vi "pharmaBot_v0.019.vi"() -> ()   [LabVIEW 2015] (continued)
            n1468 = call "get_XYZ.vi"("Actuator cluster in"=w1988) -> ("X pos (steps)"=w1996:i32, "Y pos (steps)"=w1995:i32, "Z pos (steps)"=w1994:i32)  [unwired: 10 in, 2 out]
            n1469 = Build Array(w1996, w1995, w1994) -> (w1993:i32[])
            n1470 = flat-sequence {
              tunnel: w1993 -> [w2006]
              tunnel: w1989 -> [w2005]
              frame #0 {
                n1471 = local read "location above baths"() -> (w2004:bool)
                n1472 = local read "wash bath location"() -> (w2002:bool)
                n1473 = local read "cleaning bath location"() -> (w2003:bool)
                n1474 = case shown="True" w2004 {
                  tunnel: w2006 -> [_ w2015]
                  tunnel: w2005 -> [_ w2016]
                  frame False {
                  }
                  frame True {
                    n1475 = case shown="\"manipulator 1\", Default" w2016 {
                      tunnel: w2015 -> [w2017 w2018]
                      frame "manipulator 1", Default {
                        n1476 = local write "loc above baths 1"(w2017) -> ()
                      }
                      frame "manipulator 2" {
                        n1477 = local write "loc above baths 2"(w2018) -> ()
                      }
                    }
                  }
                }
                n1478 = case shown="True" w2003 {
                  tunnel: w2006 -> [_ w2011]
                  tunnel: w2005 -> [_ w2012]
                  frame False {
                  }
                  frame True {
                    n1479 = case shown="\"manipulator 2\"" w2012 {
                      tunnel: w2011 -> [w2013 w2014]
                      frame "manipulator 1", Default {
                        n1480 = local write "cleaning bath loc 1"(w2013) -> ()
                      }
                      frame "manipulator 2" {
                        n1481 = local write "cleaning bath loc 2"(w2014) -> ()
                      }
                    }
                  }
                }
                n1482 = case shown="True" w2002 {
                  tunnel: w2006 -> [_ w2007]
                  tunnel: w2005 -> [_ w2008]
                  frame False {
                  }
                  frame True {
                    n1483 = case shown="\"manipulator 2\"" w2008 {
                      tunnel: w2007 -> [w2009 w2010]
                      frame "manipulator 1", Default {
                        n1484 = local write "wash bath loc 1"(w2009) -> ()
                      }
                      frame "manipulator 2" {
                        n1485 = local write "wash bath loc 2"(w2010) -> ()
                      }
                    }
                  }
                }
              }
              frame #1 {
                # "calculate \"above wash bath\" and \"above clean bath\" here\nin the future"
              }
            }
          }
        }
      }
      event "pipette autofocus": Value Change {
        n1486 = event-data() -> ("OldVal"=w2020:bool)  [unwired: 1 in, 5 out]
        n1487 = case shown="True" w2020 {
          tunnel: w2022 -> [_ w2039]
          tunnel: w2021 -> [_ w2038]
          frame False {
          }
          frame True {
            n1488 = local read "which manipulator to autofocus"() -> (w2024:T8)
            n1489 = case shown="\"manipulator 1\", Default" w2024 {
              tunnel: w2039 -> [w2076 w2081 w2083 w2085]
              tunnel: [w2075 w2080 w2082 w2084] -> w2037
              tunnel: [w2074 w2079 _ _] -> w2032
              tunnel: [w2073 w2078 _ _] -> w2031
              tunnel: [w2072 w2077 _ _] -> w2030
              frame "manipulator 1", Default {
                n1490 = local read "pipette 1 template"() -> (w2072:T10)
                n1491 = local read "found pipette 1"() -> (w2074:T10)
                n1492 = Unbundle By Name(w2076) -> ("manip 1"=w2075:refnum<vi>)
                n1493 = local read "manip 1 position"() -> (w2073:T23)
              }
              frame "manipulator 2" {
                n1494 = local read "pipette 2 template"() -> (w2077:T10)
                n1495 = local read "manip 2 position"() -> (w2078:T23)
                n1496 = Unbundle By Name(w2081) -> ("manip 2"=w2080:refnum<vi>)
                n1497 = local read "found pipette 2"() -> (w2079:T10)
              }
              frame "manipulator 3" {
                n1498 = Unbundle By Name(w2083) -> ("manip 3"=w2082:refnum<vi>)
              }
              frame "manipulator 4" {
                n1499 = Unbundle By Name(w2085) -> ("manip 4"=w2084:refnum<vi>)
              }
            }
            n1500 = call "get_screenCenter.vi"("image"=w2038) -> ("screen center (px)"=w2033:i32[])  [unwired: 10 in]
            n1501 = property class="Clust (strict)"(reference=w2037) -> (error out=w2028:errorcluster, "Value"=w2036:T25)  [unwired: 1 in, 1 out]
            n1502 = Unbundle By Name(w2036) -> ("actuator"=w2035:T26)
            n1503 = local read "pipette match score"() -> (w2034:sgl)
            n1504 = property on="tip found?" class="Bool (strict)"(error in=w2028, "Value"=FALSE ("tip found?")) -> (error out=w2027:errorcluster)  [unwired: 1 in, 1 out]
            n1505 = for {
              N: 1 -> [_]
              tunnel: w2033 -> [w2070]
              tunnel: [w2065] -> _
              tunnel: [w2066] -> _
              tunnel: w2035 -> [w2061]
              tunnel: w2027 -> [w2060]
              tunnel: w2039 -> [w2059]
              tunnel: w2024 -> [w2058]
              tunnel: w2038 -> [w2057]
              tunnel: w2030 -> [w2056]
              tunnel: w2032 -> [w2054]
              tunnel: [w2051] -> w2023
              tunnel: w2034 -> [w2048]
              tunnel: w2031 -> [w2053]
              tunnel: [w2043] -> w2025
              i -> [w2046]
              n1506 = call "Time Delay"("error in (no error)"=w2060, "Delay Time (s)"=1.0) -> ("error out"=w2063:errorcluster)  [unwired: 9 in]
              n1507 = Multiply(x=w2046, y=100) -> (x*y=w2050:i32)
              n1508 = Add(x=w2050, y=w2048) -> (x+y=w2047:sgl)
              n1509 = call "find_pipetteTip_v5.vi"("manip position"=w2053, "slice view"=w2057, "error in"=w2063, "pipette match score"=w2047, "pipette template"=w2056, "pipette in"=w2061) -> ("error out"=w2067:errorcluster, "tip found?"=w2051:bool, "screen tip location (px)"=w2052:i32[], "pipette out"=w2062:T26, "Score"=w2042:sgl, "found"=w2055:T10)
              n1510 = Subtract(x=w2070, y=w2052) -> (x-y=w2071:i32[])
              n1511 = call <vilib>:"Clear Errors.vi"("error in (no error)"=w2067) -> ("error out"=w2044:errorcluster)  [unwired: 5 in, 1 out]
              n1512 = local write "screen tip location (px)"(w2052) -> ()
              n1513 = call "camToPipette_rel_3d.vi"("which manipulator"=w2058, "transform cluster + actuator"=w2059, "rel cam (px)"=w2071) -> ("rel pipette (steps)"=w2069:dbl[])  [unwired: 8 in]
              n1514 = local write "pipette score"(w2042) -> ()
              n1515 = call "IMAQ Copy"("Image Dst"=w2054, "Image Src"=w2055) -> ("Image Dst Out"=w2043:T10)  [unwired: 4 in, 1 out]
              n1516 = To Long Integer(number=w2069) -> (32bit integer=w2068:i32[])
              n1517 = call "moveTo_rel_XY.vi"("blocking?"=TRUE, "error in"=w2044, "XYZ location (steps)"=w2068, "Actuator cluster in"=w2062) -> ("error out"=w2066:errorcluster, "Actuator cluster out"=w2065:T26)  [unwired: 6 in]
            }
            n1518 = local write "tip found?"(w2023) -> ()
            n1519 = case shown="\"manipulator 1\", Default" w2024 {
              tunnel: w2025 -> [w2040 w2041 _ _]
              frame "manipulator 1", Default {
                n1520 = local write "found pipette 1"(w2040) -> ()
              }
              frame "manipulator 2" {
                n1521 = local write "found pipette 2"(w2041) -> ()
              }
              frame "manipulator 3" {
              }
              frame "manipulator 4" {
              }
            }
          }
        }
      }
      event "send UUX": Value Change {
        n1522 = event-data() -> ("NewVal"=w2087:bool)  [unwired: 1 in, 5 out]
        n1523 = local read "Calibrate:"() -> (w2091:T8)
        n1524 = case shown="\"manipulator 1\", Default" w2091 {
          tunnel: w2092 -> [w2095 w2097 w2099 w2101]
          tunnel: [w2094 w2096 w2098 w2100] -> w2090
          frame "manipulator 1", Default {
            n1525 = Unbundle By Name(w2095) -> ("manip 1"=w2094:refnum<vi>)
          }
          frame "manipulator 2" {
            n1526 = Unbundle By Name(w2097) -> ("manip 2"=w2096:refnum<vi>)
          }
          frame "manipulator 3" {
            n1527 = Unbundle By Name(w2099) -> ("manip 3"=w2098:refnum<vi>)
          }
          frame "manipulator 4" {
            n1528 = Unbundle By Name(w2101) -> ("manip 4"=w2100:refnum<vi>)
          }
        }
        n1529 = property class="Clust (strict)"(reference=w2090) -> (error out=w2088:errorcluster, "Value"=w2089:T25)  [unwired: 1 in, 1 out]
        n1530 = Unbundle By Name(w2089) -> ("actuator.Actuator COM"=w2093:refnum<visa-resource-name>)
        n1531 = case shown="True" w2087 {
          tunnel: w2093 -> [_ w2105]
          tunnel: w2088 -> [_ w2104]
          frame False {
          }
          frame True {
            n1532 = call "sc_CommandSerial.vi"("error in (no error)"=w2104, "argument"="UUX", "Scientifica commands"=scientifica_commands."UUX", "VISA handle"=w2105) -> ()  [unwired: 4 in, 4 out]
          }
        }
      }
      event "send UUY": Value Change {
        n1533 = event-data() -> ("NewVal"=w2107:bool)  [unwired: 1 in, 5 out]
        n1534 = local read "Calibrate:"() -> (w2111:T8)
        n1535 = case shown="\"manipulator 1\", Default" w2111 {
          tunnel: w2112 -> [w2115 w2117 w2119 w2121]
          tunnel: [w2114 w2116 w2118 w2120] -> w2110
          frame "manipulator 1", Default {
            n1536 = Unbundle By Name(w2115) -> ("manip 1"=w2114:refnum<vi>)
          }
          frame "manipulator 2" {
            n1537 = Unbundle By Name(w2117) -> ("manip 2"=w2116:refnum<vi>)
          }
          frame "manipulator 3" {
            n1538 = Unbundle By Name(w2119) -> ("manip 3"=w2118:refnum<vi>)
          }
          frame "manipulator 4" {
            n1539 = Unbundle By Name(w2121) -> ("manip 4"=w2120:refnum<vi>)
          }
        }
        n1540 = property class="Clust (strict)"(reference=w2110) -> (error out=w2108:errorcluster, "Value"=w2109:T25)  [unwired: 1 in, 1 out]
        n1541 = Unbundle By Name(w2109) -> ("actuator.Actuator COM"=w2113:refnum<visa-resource-name>)
        n1542 = case shown="True" w2107 {
          tunnel: w2113 -> [_ w2125]
          tunnel: w2108 -> [_ w2124]
          frame False {
          }
          frame True {
            n1543 = call "sc_CommandSerial.vi"("error in (no error)"=w2124, "argument"="UUY", "Scientifica commands"=scientifica_commands."UUY", "VISA handle"=w2125) -> ()  [unwired: 4 in, 4 out]
          }
        }
      }
      event "send UUZ": Value Change {
        n1544 = event-data() -> ("NewVal"=w2127:bool)  [unwired: 1 in, 5 out]
        n1545 = local read "Calibrate:"() -> (w2131:T8)
        n1546 = case shown="\"manipulator 1\", Default" w2131 {
          tunnel: w2132 -> [w2135 w2137 w2139 w2141]
          tunnel: [w2134 w2136 w2138 w2140] -> w2130
          frame "manipulator 1", Default {
            n1547 = Unbundle By Name(w2135) -> ("manip 1"=w2134:refnum<vi>)
          }
          frame "manipulator 2" {
            n1548 = Unbundle By Name(w2137) -> ("manip 2"=w2136:refnum<vi>)
          }
          frame "manipulator 3" {
            n1549 = Unbundle By Name(w2139) -> ("manip 3"=w2138:refnum<vi>)
          }
          frame "manipulator 4" {
            n1550 = Unbundle By Name(w2141) -> ("manip 4"=w2140:refnum<vi>)
          }
        }
        n1551 = property class="Clust (strict)"(reference=w2130) -> (error out=w2128:errorcluster, "Value"=w2129:T25)  [unwired: 1 in, 1 out]
        n1552 = Unbundle By Name(w2129) -> ("actuator.Actuator COM"=w2133:refnum<visa-resource-name>)
        n1553 = case shown="True" w2127 {
          tunnel: w2133 -> [_ w2145]
          tunnel: w2128 -> [_ w2144]
          frame False {
          }
          frame True {
            n1554 = call "sc_CommandSerial.vi"("error in (no error)"=w2144, "argument"="UUZ", "Scientifica commands"=scientifica_commands."UUZ", "VISA handle"=w2145) -> ()  [unwired: 4 in, 4 out]
          }
        }
      }
      event "set safe space": Value Change {
        n1555 = event-data() -> ("NewVal"=w2148:bool)  [unwired: 1 in, 5 out]
        n1556 = case shown="True" w2148 {
          tunnel: w2147 -> [_ w2154]
          frame False {
          }
          frame True {
            n1557 = local read "Calibrate:"() -> (w2156:T8)
            n1558 = case shown="\"manipulator 4\"" w2156 {
              tunnel: w2154 -> [w2161 w2163 w2165 w2167]
              tunnel: [w2160 w2162 w2164 w2166] -> w2153
              frame "manipulator 1", Default {
                n1559 = Unbundle By Name(w2161) -> ("manip 1"=w2160:refnum<vi>)
              }
              frame "manipulator 2" {
                n1560 = Unbundle By Name(w2163) -> ("manip 2"=w2162:refnum<vi>)
              }
              frame "manipulator 3" {
                n1561 = Unbundle By Name(w2165) -> ("manip 3"=w2164:refnum<vi>)
              }
              frame "manipulator 4" {
                n1562 = Unbundle By Name(w2167) -> ("manip 4"=w2166:refnum<vi>)
              }
            }
            n1563 = property class="Clust (strict)"(reference=w2153) -> (reference out=w2152:refnum<vi>, "Value"=w2151:T25)  [unwired: 1 in, 1 out]
            n1564 = Unbundle By Name(w2151) -> ("actuator"=w2150:T26)
            n1565 = call "get_XYZ.vi"("Actuator cluster in"=w2150) -> ("X pos (steps)"=w2159:i32, "Y pos (steps)"=w2158:i32, "Z pos (steps)"=w2157:i32)  [unwired: 10 in, 2 out]
            n1566 = Build Array(w2159, w2158, w2157) -> (w2149:i32[])
            n1567 = Bundle By Name(cluster=w2151, "safe space (steps)"=w2149) -> (w2155:T25)
            n1568 = property class="Clust (strict)"(reference=w2152, "Value"=w2155) -> ()  [unwired: 1 in, 2 out]
          }
        }
      }
      event "go to safe space": Value Change {
        n1569 = event-data() -> ("NewVal"=w2171:bool)  [unwired: 1 in, 5 out]
        n1570 = case shown="True" w2171 {
          tunnel: w2170 -> [_ w2178]
          tunnel: w2169 -> [_ w2175]
          frame False {
          }
          frame True {
            n1571 = local read "Calibrate:"() -> (w2176:T8)
            n1572 = case shown="\"manipulator 4\"" w2176 {
              tunnel: w2175 -> [w2180 w2182 w2184 w2186]
              tunnel: [w2179 w2181 w2183 w2185] -> w2174
              frame "manipulator 1", Default {
                n1573 = Unbundle By Name(w2180) -> ("manip 1"=w2179:refnum<vi>)
              }
              frame "manipulator 2" {
                n1574 = Unbundle By Name(w2182) -> ("manip 2"=w2181:refnum<vi>)
              }
              frame "manipulator 3" {
                n1575 = Unbundle By Name(w2184) -> ("manip 3"=w2183:refnum<vi>)
              }
              frame "manipulator 4" {
                n1576 = Unbundle By Name(w2186) -> ("manip 4"=w2185:refnum<vi>)
              }
            }
            n1577 = property class="Clust (strict)"(reference=w2174) -> ("Value"=w2173:T25)  [unwired: 1 in, 2 out]
            n1578 = Unbundle By Name(w2173) -> ("safe space (steps)"=w2172:i32[])
            n1579 = call "move manipulator abs xyz.vi"("blocking?"=TRUE, "which manipulator"=w2176, "transform cluster + actuator"=w2175, "positions"=w2178, "location (steps)"=w2172) -> ()  [unwired: 6 in, 1 out]
          }
        }
      }
      event "zero stage", "zero stage 2", "zero stage 3": Value Change {
        n1580 = event-data() -> ("NewVal"=w2194:bool)  [unwired: 1 in, 5 out]
        n1581 = case shown="True" w2194 {
          tunnel: w2193 -> [_ w2200]
          tunnel: w2192 -> [_ w2198]
          tunnel: w2191 -> [_ w2203]
          tunnel: w2190 -> [_ _]
          tunnel: w2189 -> [_ w2201]
          tunnel: w2188 -> [_ w2199]
          frame False {
          }
          frame True {
            n1582 = Unbundle By Name(w2198) -> ("current stage pos (steps)"=w2197:refnum<vi>)
            n1583 = Unbundle By Name(w2200) -> ("s"=w2206:refnum<vi>)
            n1584 = property class="Clust (strict)"(reference=w2206) -> ("Value"=w2205:T25)  [unwired: 1 in, 2 out]
            n1585 = property class="Arr (strict)"(reference=w2197) -> ("Value"=w2196:i32[])  [unwired: 1 in, 2 out]
            n1586 = Unbundle By Name(w2205) -> ("actuator"=w2204:T26)
            n1587 = call "updateCellPositionsBasedOnNewStageZero.vi"("preZeroStageCooridinates"=w2196, "transform cluster + actuator"=w2200, "common cluster"=w2199) -> ("error out"=w2195:errorcluster)  [unwired: 8 in]
            n1588 = disable-structure shown="Disabled" {
              disable-tunnel: w2198 -> [w2214 _]
              disable-tunnel: w2203 -> [w2212 _]
              disable-tunnel: [w2209 w2215] -> w2202
              disable-tunnel: w2201 -> [w2208 _]
              disable-tunnel: w2195 -> [w2207 w2215]
              frame Disabled {
                n1589 = Unbundle By Name(w2214) -> ("current stage pos (steps)"=w2213:refnum<vi>)
                n1590 = property class="Arr (strict)"(reference=w2213) -> ("Value"=w2211:i32[])  [unwired: 1 in, 2 out]
                n1591 = call "updateJumperPositionsBasedOnNewStageZero.vi"("error in"=w2207, "preZeroStageCooridinates"=w2211, "JumperPositions"=w2212) -> ("error out"=w2210:errorcluster)  [unwired: 8 in]
                n1592 = call "updateBathPositionsBasedOnNewStageZero_v02.vi"("error in"=w2210, "preZeroStageCooridinates"=w2211, "individual controls in"=w2208) -> ("error out"=w2209:errorcluster)  [unwired: 8 in]
              }
              frame Enabled {
              }
            }
            n1593 = call "zero actuator.vi"("error in"=w2202, "actuator in"=w2204) -> ()  [unwired: 8 in, 2 out]
          }
        }
      }
      event "zero stage 6", "zero stage 5", "zero stage 4": Value Change {
        n1594 = event-data() -> ("NewVal"=w2223:bool)  [unwired: 1 in, 5 out]
        n1595 = case shown="True" w2223 {
          tunnel: w2222 -> [_ w2224]
          tunnel: w2221 -> [_ w2226]
          tunnel: w2220 -> [_ w2229]
          tunnel: w2219 -> [_ _]
          tunnel: w2218 -> [_ w2227]
          tunnel: w2217 -> [_ w2225]
          frame False {
          }
          frame True {
            n1596 = disable-structure shown="Disabled" {
              disable-tunnel: w2226 -> [w2236 _]
              disable-tunnel: w2229 -> [w2243 _]
              disable-tunnel: [w2240 _] -> w2228
              disable-tunnel: w2227 -> [w2239 _]
              disable-tunnel: w2225 -> [w2235 _]
              disable-tunnel: w2224 -> [w2234 _]
              frame Disabled {
                n1597 = Unbundle By Name(w2236) -> ("current stage pos (steps)"=w2237:refnum<vi>)
                n1598 = Unbundle By Name(w2236) -> ("current stage pos (steps)"=w2244:refnum<vi>)
                n1599 = property class="Arr (strict)"(reference=w2237) -> ("Value"=w2238:i32[])  [unwired: 1 in, 2 out]
                n1600 = property class="Arr (strict)"(reference=w2244) -> ("Value"=w2242:i32[])  [unwired: 1 in, 2 out]
                n1601 = call "updateCellPositionsBasedOnNewStageZero.vi"("preZeroStageCooridinates"=w2238, "transform cluster + actuator"=w2234, "common cluster"=w2235) -> ("error out"=w2233:errorcluster)  [unwired: 8 in]
                n1602 = call "updateJumperPositionsBasedOnNewStageZero.vi"("error in"=w2233, "preZeroStageCooridinates"=w2242, "JumperPositions"=w2243) -> ("error out"=w2241:errorcluster)  [unwired: 8 in]
                n1603 = call "updateBathPositionsBasedOnNewStageZero_v02.vi"("error in"=w2241, "preZeroStageCooridinates"=w2242, "individual controls in"=w2239) -> ("error out"=w2240:errorcluster)  [unwired: 8 in]
              }
              frame Enabled {
              }
            }
            n1604 = Unbundle By Name(w2224) -> ("s"=w2232:refnum<vi>)
            n1605 = property class="Clust (strict)"(reference=w2232) -> ("Value"=w2231:T25)  [unwired: 1 in, 2 out]
            n1606 = Unbundle By Name(w2231) -> ("actuator"=w2230:T26)
            n1607 = call "zero actuator.vi"("error in"=w2228, "actuator in"=w2230) -> ()  [unwired: 8 in, 2 out]
          }
        }
      }
      event "Zero Pipette 1", "Zero Pipette 2": Value Change {
        # "Pipette Adjustment (update other locations)\nie altering the zero location after error check"
        n1608 = event-data() -> ("NewVal"=w2250:bool)  [unwired: 1 in, 5 out]
        n1609 = case shown="True" w2250 {
          tunnel: w2249 -> [_ w2252]
          tunnel: w2248 -> [_ w2253]
          tunnel: w2247 -> [_ w2255]
          tunnel: w2246 -> [_ w2251]
          frame False {
          }
          frame True {
            n1610 = local read "Calibrate:"() -> (w2265:T8)
            n1611 = case shown="\"manipulator 1\", Default" w2265 {
              tunnel: w2252 -> [w2267 w2269 w2271 w2273]
              tunnel: [w2266 w2268 w2270 w2272] -> w2264
              frame "manipulator 1", Default {
                n1612 = Unbundle By Name(w2267) -> ("manip 1"=w2266:refnum<vi>)
              }
              frame "manipulator 2" {
                n1613 = Unbundle By Name(w2269) -> ("manip 2"=w2268:refnum<vi>)
              }
              frame "manipulator 3" {
                n1614 = Unbundle By Name(w2271) -> ("manip 3"=w2270:refnum<vi>)
              }
              frame "manipulator 4" {
                n1615 = Unbundle By Name(w2273) -> ("manip 4"=w2272:refnum<vi>)
              }
            }
            n1616 = Unbundle By Name(w2251) -> ("current manip 1 pos (steps)"=w2258:refnum<vi>)
            n1617 = property class="Clust (strict)"(reference=w2264) -> ("Value"=w2262:T25)  [unwired: 1 in, 2 out]
            n1618 = Unbundle By Name(w2262) -> ("actuator"=w2261:T26)
            n1619 = property class="Arr (strict)"(reference=w2258) -> ("Value"=w2257:i32[])  [unwired: 1 in, 2 out]
            n1620 = Unbundle By Name(w2261) -> ("Actuator COM"=w2260:refnum<visa-resource-name>)  [unwired: 1 out]
            n1621 = call "updateJumperPositionsBasedOnNewStageZero.vi"("preZeroStageCooridinates"=w2257, "JumperPositions"=w2253) -> ("error out"=w2256:errorcluster)  [unwired: 9 in]
            n1622 = call "updateBathPositionsBasedOnNewStageZero_v02.vi"("error in"=w2256, "preZeroStageCooridinates"=w2257, "individual controls in"=w2255) -> ("error out"=w2254:errorcluster)  [unwired: 8 in]
            n1623 = call "zero actuator.vi"("error in"=w2254, "actuator in"=w2261) -> ("error out"=w2259:errorcluster)  [unwired: 8 in, 1 out]
            n1624 = call "sc_adjustMotion.vi"("error in (no error)"=w2259, "motion"=scope_motion."fast", "VISA handle"=w2260) -> ()  [unwired: 7 in, 2 out]
          }
        }
      }
      event "Zero Pipette 3", "Zero Pipette 4": Value Change {
        # "New Pipette (don't adjust other locations)\nor Error Adjustment after large movements"
        n1625 = event-data() -> ("NewVal"=w2279:bool)  [unwired: 1 in, 5 out]
        n1626 = case shown="True" w2279 {
          tunnel: w2278 -> [_ w2281]
          tunnel: w2277 -> [_ w2282]
          tunnel: w2276 -> [_ w2284]
          tunnel: w2275 -> [_ w2280]
          frame False {
          }
          frame True {
            n1627 = local read "Calibrate:"() -> (w2291:T8)
            n1628 = case shown="\"manipulator 1\", Default" w2291 {
              tunnel: w2281 -> [w2300 w2302 w2304 w2306]
              tunnel: [w2299 w2301 w2303 w2305] -> w2290
              frame "manipulator 1", Default {
                n1629 = Unbundle By Name(w2300) -> ("manip 1"=w2299:refnum<vi>)
              }
              frame "manipulator 2" {
                n1630 = Unbundle By Name(w2302) -> ("manip 2"=w2301:refnum<vi>)
              }
              frame "manipulator 3" {
                n1631 = Unbundle By Name(w2304) -> ("manip 3"=w2303:refnum<vi>)
              }
              frame "manipulator 4" {
                n1632 = Unbundle By Name(w2306) -> ("manip 4"=w2305:refnum<vi>)
              }
            }
            n1633 = disable-structure shown="Disabled" {
              disable-tunnel: w2284 -> [w2295 _]
              disable-tunnel: [w2294 _] -> w2283
              disable-tunnel: w2282 -> [w2293 _]
              disable-tunnel: w2280 -> [w2292 _]
              frame Disabled {
                n1634 = Unbundle By Name(w2292) -> ("current manip 1 pos (steps)"=w2298:refnum<vi>)
                n1635 = property class="Arr (strict)"(reference=w2298) -> ("Value"=w2297:i32[])  [unwired: 1 in, 2 out]
                n1636 = call "updateJumperPositionsBasedOnNewStageZero.vi"("preZeroStageCooridinates"=w2297, "JumperPositions"=w2293) -> ("error out"=w2296:errorcluster)  [unwired: 9 in]
                n1637 = call "updateBathPositionsBasedOnNewStageZero_v02.vi"("error in"=w2296, "preZeroStageCooridinates"=w2297, "individual controls in"=w2295) -> ("error out"=w2294:errorcluster)  [unwired: 8 in]
              }
              frame Enabled {
              }
            }
            n1638 = property class="Clust (strict)"(reference=w2290) -> ("Value"=w2288:T25)  [unwired: 1 in, 2 out]
            n1639 = Unbundle By Name(w2288) -> ("actuator"=w2287:T26)
            n1640 = Unbundle By Name(w2287) -> ("Actuator COM"=w2286:refnum<visa-resource-name>)  [unwired: 1 out]
            n1641 = call "zero actuator.vi"("error in"=w2283, "actuator in"=w2287) -> ("error out"=w2285:errorcluster)  [unwired: 8 in, 1 out]
            n1642 = call "sc_adjustMotion.vi"("error in (no error)"=w2285, "motion"=scope_motion."fast", "VISA handle"=w2286) -> ()  [unwired: 7 in, 2 out]
          }
        }
      }
      event "go to zero": Value Change {
        n1643 = event-data() -> ("NewVal"=w2309:bool)  [unwired: 1 in, 5 out]
        n1644 = case shown="True" w2309 {
          tunnel: w2308 -> [_ w2328]
          frame False {
          }
          frame True {
            w2310 = scope_motion."slow_dualPatch" ("motion")
            w2331 = TRUE ("blocking?")
            w2330 = 0
            n1645 = Unbundle By Name(w2328) -> ("s"=w2324:refnum<vi>)
            n1646 = local read "Calibrate:"() -> (w2327:T8)
            n1647 = property class="Clust (strict)"(reference=w2324) -> ("Value"=w2323:T25)  [unwired: 1 in, 2 out]
            n1648 = case shown="\"manipulator 1\", Default" w2327 {
              tunnel: w2328 -> [w2333 w2335 w2337 w2339]
              tunnel: [w2332 w2334 w2336 w2338] -> w2326
              frame "manipulator 1", Default {
                n1649 = Unbundle By Name(w2333) -> ("manip 1"=w2332:refnum<vi>)
              }
              frame "manipulator 2" {
                n1650 = Unbundle By Name(w2335) -> ("manip 2"=w2334:refnum<vi>)
              }
              frame "manipulator 3" {
                n1651 = Unbundle By Name(w2337) -> ("manip 3"=w2336:refnum<vi>)
              }
              frame "manipulator 4" {
                n1652 = Unbundle By Name(w2339) -> ("manip 4"=w2338:refnum<vi>)
              }
            }
            n1653 = Unbundle By Name(w2323) -> ("actuator"=w2313:T26)
            n1654 = Unbundle By Name(w2313) -> ("Actuator COM"=w2312:refnum<visa-resource-name>)  [unwired: 1 out]
            n1655 = property class="Clust (strict)"(reference=w2326) -> (error out=w2316:errorcluster, "Value"=w2325:T25)  [unwired: 1 in, 1 out]
            n1656 = Build Array(w2330, w2330, w2330) -> (w2329:i32[])
            n1657 = Unbundle By Name(w2325) -> ("actuator"=w2321:T26)
            n1658 = Unbundle By Name(w2321) -> ("Actuator COM"=w2319:refnum<visa-resource-name>)  [unwired: 1 out]
            n1659 = call "sc_adjustMotion.vi"("error in (no error)"=w2316, "motion"=scope_motion."slow_dualPatch", "VISA handle"=w2312) -> ("error out"=w2315:errorcluster)  [unwired: 7 in, 1 out]
            n1660 = call "moveTo_abs_XYZ.vi"("blocking?"=w2331, "error in"=w2315, "XYZ location (steps)"=w2329, "Actuator cluster in"=w2313) -> ("error out"=w2318:errorcluster)  [unwired: 6 in, 1 out]
            n1661 = call "sc_adjustMotion.vi"("error in (no error)"=w2318, "motion"=scope_motion."fast", "VISA handle"=w2319) -> ("error out"=w2317:errorcluster)  [unwired: 7 in, 1 out]
            n1662 = call "moveTo_abs_XYZ.vi"("blocking?"=w2331, "error in"=w2317, "XYZ location (steps)"=w2329, "Actuator cluster in"=w2321) -> ("error out"=w2320:errorcluster)  [unwired: 6 in, 1 out]
            n1663 = call "sc_adjustMotion.vi"("error in (no error)"=w2320, "motion"=w2310, "VISA handle"=w2319) -> ("error out"=w2311:errorcluster)  [unwired: 7 in, 1 out]
            n1664 = call "sc_adjustMotion.vi"("error in (no error)"=w2311, "motion"=w2310, "VISA handle"=w2312) -> ()  [unwired: 7 in, 2 out]
          }
        }
      }
      event "Raise Manipulator": Value Change {
        n1665 = event-data() -> ("NewVal"=w2343:bool)  [unwired: 1 in, 5 out]
        n1666 = case shown="True" w2343 {
          tunnel: w2342 -> [_ w2345]
          tunnel: w2341 -> [_ w2346]
          frame False {
          }
          frame True {
            w2358 = 0
            n1667 = local read "Calibrate:"() -> (w2348:T8)
            n1668 = case shown="\"manipulator 1\", Default" w2348 {
              tunnel: w2345 -> [w2361 w2363 w2365 w2367]
              tunnel: [w2360 w2362 w2364 w2366] -> w2357
              frame "manipulator 1", Default {
                n1669 = Unbundle By Name(w2361) -> ("manip 1"=w2360:refnum<vi>)
              }
              frame "manipulator 2" {
                n1670 = Unbundle By Name(w2363) -> ("manip 2"=w2362:refnum<vi>)
              }
              frame "manipulator 3" {
                n1671 = Unbundle By Name(w2365) -> ("manip 3"=w2364:refnum<vi>)
              }
              frame "manipulator 4" {
                n1672 = Unbundle By Name(w2367) -> ("manip 4"=w2366:refnum<vi>)
              }
            }
            n1673 = property class="Clust (strict)"(reference=w2357) -> (error out=w2354:errorcluster, "Value"=w2356:T25)  [unwired: 1 in, 1 out]
            n1674 = Build Array(w2358, w2358, -10000 ("element")) -> (w2347:i32[])
            n1675 = Unbundle By Name(w2356) -> ("actuator"=w2352:T26)  [unwired: 1 out]
            n1676 = Unbundle By Name(w2352) -> ("Actuator COM"=w2349:refnum<visa-resource-name>)  [unwired: 1 out]
            n1677 = call "sc_adjustMotion.vi"("error in (no error)"=w2354, "motion"=scope_motion."fast", "VISA handle"=w2349) -> ("error out"=w2353:errorcluster)  [unwired: 7 in, 1 out]
            n1678 = call "move manipulator rel.vi"("blocking?"=TRUE, "which manipulator"=w2348, "error in (no error)"=w2353, "transform cluster + actuator"=w2345, "positions"=w2346, "location (steps)"=w2347) -> ("error out"=w2350:errorcluster)  [unwired: 5 in]
            n1679 = call "sc_adjustMotion.vi"("error in (no error)"=w2350, "motion"=scope_motion."slow_dualPatch", "VISA handle"=w2349) -> ()  [unwired: 7 in, 2 out]
          }
        }
      }
      event "Raise Stage 300 uM", "Lower Stage 300 uM": Value Change {
        n1680 = event-data() -> ("CtlRef"=w2379:refnum<vi>, "NewVal"=w2382:bool)  [unwired: 1 in, 4 out]
        n1681 = property class="Bool (strict)"(reference=w2379) -> ("Label.Text"=w2378:string)  [unwired: 1 in, 2 out]
        n1682 = Equal?(x=w2378, y="Raise Stage 300 uM") -> (x = y?=w2373:bool)
        n1683 = Select(t=1.0, s=w2373, f=-1.0) -> (s? t:f=w2370:dbl)
        n1684 = Multiply(x=300 ("element"), y=75.3) -> (x*y=w2374:dbl)
        n1685 = Multiply(x=w2374, y=w2370) -> (x*y=w2369:dbl)
        n1686 = case shown="True" w2382 {
          tunnel: w2381 -> [_ w2385]
          tunnel: w2380 -> [_ w2386]
          tunnel: w2369 -> [_ w2384]
          frame False {
          }
          frame True {
            w2397 = 0
            n1687 = Unbundle By Name(w2385) -> ("s"=w2396:refnum<vi>)
            n1688 = property class="Clust (strict)"(reference=w2396) -> (error out=w2393:errorcluster, "Value"=w2395:T25)  [unwired: 1 in, 1 out]
            n1689 = To Long Integer(number=w2384) -> (32bit integer=w2383:i32)
            n1690 = Build Array(w2397, w2397, w2383) -> (w2387:i32[])
            n1691 = Unbundle By Name(w2395) -> ("actuator"=w2391:T26)  [unwired: 1 out]
            n1692 = Unbundle By Name(w2391) -> ("Actuator COM"=w2388:refnum<visa-resource-name>)  [unwired: 1 out]
            n1693 = call "sc_adjustMotion.vi"("error in (no error)"=w2393, "motion"=scope_motion."slow_dualPatch", "VISA handle"=w2388) -> ("error out"=w2392:errorcluster)  [unwired: 7 in, 1 out]
            n1694 = call "move stage rel.vi"("blocking?"=TRUE, "error in (no error)"=w2392, "transform cluster + actuator"=w2385, "positions"=w2386, "rel move (steps)"=w2387) -> ("error out"=w2389:errorcluster)  [unwired: 6 in]
            n1695 = call "sc_adjustMotion.vi"("error in (no error)"=w2389, "motion"=scope_motion."slow_dualPatch", "VISA handle"=w2388) -> ()  [unwired: 7 in, 2 out]
          }
        }
      }
      event "MZ Dn", "MZ Up", "MX Up", "MX Dn", "MY Dn", "MY Up", "SZ Dn", "SZ Up", "SX Up", "SX Dn", "SY Dn", "SY Up": Value Change {
        n1696 = event-data() -> ("CtlRef"=w2405:refnum<vi>)  [unwired: 1 in, 5 out]
        n1697 = property class="Bool (strict)"(reference=w2405) -> ("Label.Text"=w2408:string)  [unwired: 1 in, 2 out]
        n1698 = String Subset(string=w2408, offset (0)=0, length (rest)=1 ("length (rest)")) -> (substring=w2412:string)
        n1699 = Equal?(x="M", y=w2412) -> (x = y?=w2410:bool)
        n1700 = case shown="False" w2410 {
          tunnel: [w2418 w2419] -> w2409
          frame False {
            n1701 = local read "Stage Button Step Size (um)"() -> (w2418:dbl)
          }
          frame True {
            n1702 = local read "Manipulator Button Step Size (um)"() -> (w2419:dbl)
          }
        }
        n1703 = Multiply(x=10.0, y=w2409) -> (x*y=w2400:dbl)
        n1704 = case shown="\"SZ Up\"" w2408 {
          tunnel: w2417 -> [_ w2426 w2443 w2461 w2478 w2496 w2516 w2536 w2554 w2573 w2591 w2610 w2628]
          tunnel: w2416 -> [_ w2427 w2444 w2462 w2479 w2497 w2517 w2537 w2555 w2574 w2592 w2611 w2629]
          tunnel: w2400 -> [_ w2425 w2442 w2460 w2477 w2493 w2512 w2535 w2553 w2572 w2590 w2609 w2627]
          tunnel: [errorcluster {"status"=FALSE, "code"=0, "source"=""} ("error out") w2422 w2439 w2457 w2474 w2494 w2513 w2532 w2550 w2571 w2589 w2608 w2626] -> w2407
          tunnel: T8."manipulator 1" ("which manipulator") -> [_ _ _ _ _ _ _ w2531 w2549 w2568 w2586 w2605 w2623]
          tunnel: 7.53 ("y") -> [_ _ _ _ _ w2491 w2510 _ _ _ _ _ _]
          frame "False", Default {
          }
          frame "SX Up" {
            w2423 = 0
            n1705 = Unbundle By Name(w2426) -> ("s"=w2437:refnum<vi>)
            n1706 = property class="Clust (strict)"(reference=w2437) -> (error out=w2434:errorcluster, "Value"=w2436:T25)  [unwired: 1 in, 1 out]
            n1707 = Unbundle By Name(w2436) -> ("actuator"=w2432:T26)  [unwired: 1 out]
            n1708 = Unbundle By Name(w2432) -> ("Actuator COM"=w2429:refnum<visa-resource-name>)  [unwired: 1 out]
            n1709 = Negate(x=w2425) -> (-x=w2421:dbl)
            n1710 = call "sc_adjustMotion.vi"("error in (no error)"=w2434, "motion"=scope_motion."slow_dualPatch", "VISA handle"=w2429) -> ("error out"=w2433:errorcluster)  [unwired: 7 in, 1 out]
            n1711 = To Long Integer(number=w2421) -> (32bit integer=w2424:i32)
            n1712 = Build Array(w2424, w2423, w2423) -> (w2428:i32[])
            n1713 = call "move stage rel.vi"("blocking?"=TRUE, "error in (no error)"=w2433, "transform cluster + actuator"=w2426, "positions"=w2427, "rel move (steps)"=w2428) -> ("error out"=w2430:errorcluster)  [unwired: 6 in]
            n1714 = call "sc_adjustMotion.vi"("error in (no error)"=w2430, "motion"=scope_motion."slow_dualPatch", "VISA handle"=w2429) -> ("error out"=w2422:errorcluster)  [unwired: 7 in, 1 out]
          }
          frame "SX Dn" {
            w2440 = 0
            n1715 = Unbundle By Name(w2443) -> ("s"=w2454:refnum<vi>)
            n1716 = property class="Clust (strict)"(reference=w2454) -> (error out=w2451:errorcluster, "Value"=w2453:T25)  [unwired: 1 in, 1 out]
            n1717 = Unbundle By Name(w2453) -> ("actuator"=w2449:T26)  [unwired: 1 out]
            n1718 = Unbundle By Name(w2449) -> ("Actuator COM"=w2446:refnum<visa-resource-name>)  [unwired: 1 out]
            n1719 = call "sc_adjustMotion.vi"("error in (no error)"=w2451, "motion"=scope_motion."slow_dualPatch", "VISA handle"=w2446) -> ("error out"=w2450:errorcluster)  [unwired: 7 in, 1 out]
            n1720 = To Long Integer(number=w2442) -> (32bit integer=w2441:i32)
            n1721 = Build Array(w2441, w2440, w2440) -> (w2445:i32[])
            n1722 = call "move stage rel.vi"("blocking?"=TRUE, "error in (no error)"=w2450, "transform cluster + actuator"=w2443, "positions"=w2444, "rel move (steps)"=w2445) -> ("error out"=w2447:errorcluster)  [unwired: 6 in]
            n1723 = call "sc_adjustMotion.vi"("error in (no error)"=w2447, "motion"=scope_motion."slow_dualPatch", "VISA handle"=w2446) -> ("error out"=w2439:errorcluster)  [unwired: 7 in, 1 out]
          }
          frame "SY Up" {
            w2458 = 0
            n1724 = Unbundle By Name(w2461) -> ("s"=w2472:refnum<vi>)
            n1725 = property class="Clust (strict)"(reference=w2472) -> (error out=w2469:errorcluster, "Value"=w2471:T25)  [unwired: 1 in, 1 out]
            n1726 = Unbundle By Name(w2471) -> ("actuator"=w2467:T26)  [unwired: 1 out]
            n1727 = Unbundle By Name(w2467) -> ("Actuator COM"=w2464:refnum<visa-resource-name>)  [unwired: 1 out]
            n1728 = Negate(x=w2460) -> (-x=w2456:dbl)
            n1729 = call "sc_adjustMotion.vi"("error in (no error)"=w2469, "motion"=scope_motion."slow_dualPatch", "VISA handle"=w2464) -> ("error out"=w2468:errorcluster)  [unwired: 7 in, 1 out]
            n1730 = To Long Integer(number=w2456) -> (32bit integer=w2459:i32)
            n1731 = Build Array(w2458, w2459, w2458) -> (w2463:i32[])
            n1732 = call "move stage rel.vi"("blocking?"=TRUE, "error in (no error)"=w2468, "transform cluster + actuator"=w2461, "positions"=w2462, "rel move (steps)"=w2463) -> ("error out"=w2465:errorcluster)  [unwired: 6 in]
            n1733 = call "sc_adjustMotion.vi"("error in (no error)"=w2465, "motion"=scope_motion."slow_dualPatch", "VISA handle"=w2464) -> ("error out"=w2457:errorcluster)  [unwired: 7 in, 1 out]
          }
          frame "SY Dn" {
            w2475 = 0
            n1734 = Unbundle By Name(w2478) -> ("s"=w2489:refnum<vi>)
            n1735 = property class="Clust (strict)"(reference=w2489) -> (error out=w2486:errorcluster, "Value"=w2488:T25)  [unwired: 1 in, 1 out]
            n1736 = Unbundle By Name(w2488) -> ("actuator"=w2484:T26)  [unwired: 1 out]
            n1737 = Unbundle By Name(w2484) -> ("Actuator COM"=w2481:refnum<visa-resource-name>)  [unwired: 1 out]
            n1738 = call "sc_adjustMotion.vi"("error in (no error)"=w2486, "motion"=scope_motion."slow_dualPatch", "VISA handle"=w2481) -> ("error out"=w2485:errorcluster)  [unwired: 7 in, 1 out]
            n1739 = To Long Integer(number=w2477) -> (32bit integer=w2476:i32)
            n1740 = Build Array(w2475, w2476, w2475) -> (w2480:i32[])
            n1741 = call "move stage rel.vi"("blocking?"=TRUE, "error in (no error)"=w2485, "transform cluster + actuator"=w2478, "positions"=w2479, "rel move (steps)"=w2480) -> ("error out"=w2482:errorcluster)  [unwired: 6 in]
            n1742 = call "sc_adjustMotion.vi"("error in (no error)"=w2482, "motion"=scope_motion."slow_dualPatch", "VISA handle"=w2481) -> ("error out"=w2474:errorcluster)  [unwired: 7 in, 1 out]
          }
          frame "SZ Up" {
            w2508 = 0
            n1743 = Unbundle By Name(w2496) -> ("s"=w2507:refnum<vi>)
            n1744 = property class="Clust (strict)"(reference=w2507) -> (error out=w2504:errorcluster, "Value"=w2506:T25)  [unwired: 1 in, 1 out]
            n1745 = Multiply(x=w2493, y=w2491) -> (x*y=w2492:dbl)
            n1746 = Unbundle By Name(w2506) -> ("actuator"=w2502:T26)  [unwired: 1 out]
            n1747 = Unbundle By Name(w2502) -> ("Actuator COM"=w2499:refnum<visa-resource-name>)  [unwired: 1 out]
            n1748 = call "sc_adjustMotion.vi"("error in (no error)"=w2504, "motion"=scope_motion."slow", "VISA handle"=w2499) -> ("error out"=w2503:errorcluster)  [unwired: 7 in, 1 out]
            n1749 = To Long Integer(number=w2492) -> (32bit integer=w2495:i32)
            n1750 = Build Array(w2508, w2508, w2495) -> (w2498:i32[])
            n1751 = call "move stage rel.vi"("blocking?"=TRUE, "error in (no error)"=w2503, "transform cluster + actuator"=w2496, "positions"=w2497, "rel move (steps)"=w2498) -> ("error out"=w2500:errorcluster)  [unwired: 6 in]
            n1752 = call "sc_adjustMotion.vi"("error in (no error)"=w2500, "motion"=scope_motion."slow_dualPatch", "VISA handle"=w2499) -> ("error out"=w2494:errorcluster)  [unwired: 7 in, 1 out]
          }
          frame "SZ Dn" {
            w2528 = 0
            n1753 = Unbundle By Name(w2516) -> ("s"=w2527:refnum<vi>)
            n1754 = property class="Clust (strict)"(reference=w2527) -> (error out=w2524:errorcluster, "Value"=w2526:T25)  [unwired: 1 in, 1 out]
            n1755 = Multiply(x=w2512, y=w2510) -> (x*y=w2511:dbl)
            n1756 = Unbundle By Name(w2526) -> ("actuator"=w2522:T26)  [unwired: 1 out]
            n1757 = Unbundle By Name(w2522) -> ("Actuator COM"=w2519:refnum<visa-resource-name>)  [unwired: 1 out]
            n1758 = Negate(x=w2511) -> (-x=w2514:dbl)
            n1759 = call "sc_adjustMotion.vi"("error in (no error)"=w2524, "motion"=scope_motion."slow", "VISA handle"=w2519) -> ("error out"=w2523:errorcluster)  [unwired: 7 in, 1 out]
            n1760 = To Long Integer(number=w2514) -> (32bit integer=w2515:i32)
            n1761 = Build Array(w2528, w2528, w2515) -> (w2518:i32[])
            n1762 = call "move stage rel.vi"("blocking?"=TRUE, "error in (no error)"=w2523, "transform cluster + actuator"=w2516, "positions"=w2517, "rel move (steps)"=w2518) -> ("error out"=w2520:errorcluster)  [unwired: 6 in]
            n1763 = call "sc_adjustMotion.vi"("error in (no error)"=w2520, "motion"=scope_motion."slow_dualPatch", "VISA handle"=w2519) -> ("error out"=w2513:errorcluster)  [unwired: 7 in, 1 out]
          }
          frame "MX Up" {
            w2533 = 0
            n1764 = Unbundle By Name(w2536) -> ("manip 1"=w2547:refnum<vi>)
            n1765 = property class="Clust (strict)"(reference=w2547) -> (error out=w2544:errorcluster, "Value"=w2546:T25)  [unwired: 1 in, 1 out]
            n1766 = Unbundle By Name(w2546) -> ("actuator"=w2542:T26)  [unwired: 1 out]
            n1767 = Unbundle By Name(w2542) -> ("Actuator COM"=w2539:refnum<visa-resource-name>)  [unwired: 1 out]
            n1768 = Negate(x=w2535) -> (-x=w2530:dbl)
            n1769 = call "sc_adjustMotion.vi"("error in (no error)"=w2544, "motion"=scope_motion."slow_dualPatch", "VISA handle"=w2539) -> ("error out"=w2543:errorcluster)  [unwired: 7 in, 1 out]
            n1770 = To Long Integer(number=w2530) -> (32bit integer=w2534:i32)
            n1771 = Build Array(w2534, w2533, w2533) -> (w2538:i32[])
            n1772 = call "move manipulator rel.vi"("blocking?"=TRUE, "which manipulator"=w2531, "error in (no error)"=w2543, "transform cluster + actuator"=w2536, "positions"=w2537, "location (steps)"=w2538) -> ("error out"=w2540:errorcluster)  [unwired: 5 in]
            n1773 = call "sc_adjustMotion.vi"("error in (no error)"=w2540, "motion"=scope_motion."slow_dualPatch", "VISA handle"=w2539) -> ("error out"=w2532:errorcluster)  [unwired: 7 in, 1 out]
          }
          frame "MX Dn" {
            w2551 = 0
            n1774 = Unbundle By Name(w2554) -> ("manip 1"=w2565:refnum<vi>)
            n1775 = property class="Clust (strict)"(reference=w2565) -> (error out=w2562:errorcluster, "Value"=w2564:T25)  [unwired: 1 in, 1 out]
            n1776 = Unbundle By Name(w2564) -> ("actuator"=w2560:T26)  [unwired: 1 out]
            n1777 = Unbundle By Name(w2560) -> ("Actuator COM"=w2557:refnum<visa-resource-name>)  [unwired: 1 out]
            n1778 = call "sc_adjustMotion.vi"("error in (no error)"=w2562, "motion"=scope_motion."slow_dualPatch", "VISA handle"=w2557) -> ("error out"=w2561:errorcluster)  [unwired: 7 in, 1 out]
            n1779 = To Long Integer(number=w2553) -> (32bit integer=w2552:i32)
            n1780 = Build Array(w2552, w2551, w2551) -> (w2556:i32[])
            n1781 = call "move manipulator rel.vi"("blocking?"=TRUE, "which manipulator"=w2549, "error in (no error)"=w2561, "transform cluster + actuator"=w2554, "positions"=w2555, "location (steps)"=w2556) -> ("error out"=w2558:errorcluster)  [unwired: 5 in]
            n1782 = call "sc_adjustMotion.vi"("error in (no error)"=w2558, "motion"=scope_motion."slow_dualPatch", "VISA handle"=w2557) -> ("error out"=w2550:errorcluster)  [unwired: 7 in, 1 out]
          }
          frame "MY Up" {
            w2570 = 0
            n1783 = Unbundle By Name(w2573) -> ("manip 1"=w2584:refnum<vi>)
            n1784 = property class="Clust (strict)"(reference=w2584) -> (error out=w2581:errorcluster, "Value"=w2583:T25)  [unwired: 1 in, 1 out]
            n1785 = Unbundle By Name(w2583) -> ("actuator"=w2579:T26)  [unwired: 1 out]
            n1786 = Unbundle By Name(w2579) -> ("Actuator COM"=w2576:refnum<visa-resource-name>)  [unwired: 1 out]
            n1787 = Negate(x=w2572) -> (-x=w2567:dbl)
            n1788 = call "sc_adjustMotion.vi"("error in (no error)"=w2581, "motion"=scope_motion."slow_dualPatch", "VISA handle"=w2576) -> ("error out"=w2580:errorcluster)  [unwired: 7 in, 1 out]
            n1789 = To Long Integer(number=w2567) -> (32bit integer=w2569:i32)
            n1790 = Build Array(w2570, w2569, w2570) -> (w2575:i32[])
            n1791 = call "move manipulator rel.vi"("blocking?"=TRUE, "which manipulator"=w2568, "error in (no error)"=w2580, "transform cluster + actuator"=w2573, "positions"=w2574, "location (steps)"=w2575) -> ("error out"=w2577:errorcluster)  [unwired: 5 in]
            n1792 = call "sc_adjustMotion.vi"("error in (no error)"=w2577, "motion"=scope_motion."slow_dualPatch", "VISA handle"=w2576) -> ("error out"=w2571:errorcluster)  [unwired: 7 in, 1 out]
          }
          frame "MY Dn" {
            w2588 = 0
            n1793 = Unbundle By Name(w2591) -> ("manip 1"=w2602:refnum<vi>)
            n1794 = property class="Clust (strict)"(reference=w2602) -> (error out=w2599:errorcluster, "Value"=w2601:T25)  [unwired: 1 in, 1 out]
            n1795 = Unbundle By Name(w2601) -> ("actuator"=w2597:T26)  [unwired: 1 out]
            n1796 = Unbundle By Name(w2597) -> ("Actuator COM"=w2594:refnum<visa-resource-name>)  [unwired: 1 out]
            n1797 = call "sc_adjustMotion.vi"("error in (no error)"=w2599, "motion"=scope_motion."slow_dualPatch", "VISA handle"=w2594) -> ("error out"=w2598:errorcluster)  [unwired: 7 in, 1 out]
            n1798 = To Long Integer(number=w2590) -> (32bit integer=w2587:i32)
            n1799 = Build Array(w2588, w2587, w2588) -> (w2593:i32[])
            n1800 = call "move manipulator rel.vi"("blocking?"=TRUE, "which manipulator"=w2586, "error in (no error)"=w2598, "transform cluster + actuator"=w2591, "positions"=w2592, "location (steps)"=w2593) -> ("error out"=w2595:errorcluster)  [unwired: 5 in]
            n1801 = call "sc_adjustMotion.vi"("error in (no error)"=w2595, "motion"=scope_motion."slow_dualPatch", "VISA handle"=w2594) -> ("error out"=w2589:errorcluster)  [unwired: 7 in, 1 out]
          }
          frame "MZ Up" {
            w2606 = 0
            n1802 = Unbundle By Name(w2610) -> ("manip 1"=w2621:refnum<vi>)
            n1803 = property class="Clust (strict)"(reference=w2621) -> (error out=w2618:errorcluster, "Value"=w2620:T25)  [unwired: 1 in, 1 out]
            n1804 = Unbundle By Name(w2620) -> ("actuator"=w2616:T26)  [unwired: 1 out]
            n1805 = Unbundle By Name(w2616) -> ("Actuator COM"=w2613:refnum<visa-resource-name>)  [unwired: 1 out]
            n1806 = Negate(x=w2609) -> (-x=w2604:dbl)
            n1807 = call "sc_adjustMotion.vi"("error in (no error)"=w2618, "motion"=scope_motion."slow_dualPatch", "VISA handle"=w2613) -> ("error out"=w2617:errorcluster)  [unwired: 7 in, 1 out]
            n1808 = To Long Integer(number=w2604) -> (32bit integer=w2607:i32)
            n1809 = Build Array(w2606, w2606, w2607) -> (w2612:i32[])
            n1810 = call "move manipulator rel.vi"("blocking?"=TRUE, "which manipulator"=w2605, "error in (no error)"=w2617, "transform cluster + actuator"=w2610, "positions"=w2611, "location (steps)"=w2612) -> ("error out"=w2614:errorcluster)  [unwired: 5 in]
            n1811 = call "sc_adjustMotion.vi"("error in (no error)"=w2614, "motion"=scope_motion."slow_dualPatch", "VISA handle"=w2613) -> ("error out"=w2608:errorcluster)  [unwired: 7 in, 1 out]
          }
          frame "MZ Dn" {
            w2624 = 0
            n1812 = Unbundle By Name(w2628) -> ("manip 1"=w2639:refnum<vi>)
            n1813 = property class="Clust (strict)"(reference=w2639) -> (error out=w2636:errorcluster, "Value"=w2638:T25)  [unwired: 1 in, 1 out]
            n1814 = Unbundle By Name(w2638) -> ("actuator"=w2634:T26)  [unwired: 1 out]
            n1815 = Unbundle By Name(w2634) -> ("Actuator COM"=w2631:refnum<visa-resource-name>)  [unwired: 1 out]
            n1816 = call "sc_adjustMotion.vi"("error in (no error)"=w2636, "motion"=scope_motion."slow_dualPatch", "VISA handle"=w2631) -> ("error out"=w2635:errorcluster)  [unwired: 7 in, 1 out]
            n1817 = To Long Integer(number=w2627) -> (32bit integer=w2625:i32)
            n1818 = Build Array(w2624, w2624, w2625) -> (w2630:i32[])
            n1819 = call "move manipulator rel.vi"("blocking?"=TRUE, "which manipulator"=w2623, "error in (no error)"=w2635, "transform cluster + actuator"=w2628, "positions"=w2629, "location (steps)"=w2630) -> ("error out"=w2632:errorcluster)  [unwired: 5 in]
            n1820 = call "sc_adjustMotion.vi"("error in (no error)"=w2632, "motion"=scope_motion."slow_dualPatch", "VISA handle"=w2631) -> ("error out"=w2626:errorcluster)  [unwired: 7 in, 1 out]
          }
        }
        n1821 = call "Time Delay4"("error in (no error)"=w2407, "Delay Time (s)"=0.1) -> ("error out"=w2403:errorcluster)  [unwired: 9 in]
        n1822 = property class="Bool (strict)"(reference=w2405, error in=w2403, "Value"=FALSE) -> ()  [unwired: 2 out]
      }
      event "send Manip to XY ZERO": Value Change {
        n1823 = event-data() -> ("NewVal"=w2644:bool)  [unwired: 1 in, 5 out]
        n1824 = case shown="True" w2644 {
          tunnel: w2643 -> [_ w2645]
          tunnel: w2642 -> [_ w2646]
          frame False {
          }
          frame True {
            w2658 = 0
            n1825 = local read "Calibrate:"() -> (w2648:T8)
            n1826 = case shown="\"manipulator 1\", Default" w2648 {
              tunnel: w2645 -> [w2661 w2663 w2665 w2667]
              tunnel: [w2660 w2662 w2664 w2666] -> w2657
              frame "manipulator 1", Default {
                n1827 = Unbundle By Name(w2661) -> ("manip 1"=w2660:refnum<vi>)
              }
              frame "manipulator 2" {
                n1828 = Unbundle By Name(w2663) -> ("manip 2"=w2662:refnum<vi>)
              }
              frame "manipulator 3" {
                n1829 = Unbundle By Name(w2665) -> ("manip 3"=w2664:refnum<vi>)
              }
              frame "manipulator 4" {
                n1830 = Unbundle By Name(w2667) -> ("manip 4"=w2666:refnum<vi>)
              }
            }
            n1831 = property class="Clust (strict)"(reference=w2657) -> (error out=w2654:errorcluster, "Value"=w2656:T25)  [unwired: 1 in, 1 out]
            n1832 = Build Array(w2658, w2658) -> (w2647:i32[])
            n1833 = Unbundle By Name(w2656) -> ("actuator"=w2652:T26)  [unwired: 1 out]
            n1834 = Unbundle By Name(w2652) -> ("Actuator COM"=w2649:refnum<visa-resource-name>)  [unwired: 1 out]
            n1835 = call "sc_adjustMotion.vi"("error in (no error)"=w2654, "motion"=scope_motion."fast", "VISA handle"=w2649) -> ("error out"=w2653:errorcluster)  [unwired: 7 in, 1 out]
            n1836 = call "move manipulator abs xy.vi"("blocking?"=TRUE, "which manipulator"=w2648, "error in (no error)"=w2653, "transform cluster + actuator"=w2645, "positions"=w2646, "location (steps)"=w2647) -> ("error out"=w2650:errorcluster)  [unwired: 5 in]
            n1837 = call "sc_adjustMotion.vi"("error in (no error)"=w2650, "motion"=scope_motion."slow_dualPatch", "VISA handle"=w2649) -> ()  [unwired: 7 in, 2 out]
          }
        }
      }
      event "send Manip to Approach Line": Value Change {
        n1838 = event-data() -> ("NewVal"=w2671:bool)  [unwired: 1 in, 5 out]
        n1839 = case shown="True" w2671 {
          tunnel: w2669 -> [_ w2680]
          tunnel: w2670 -> [_ w2681]
          frame False {
          }
          frame True {
            w2674 = -10000
            n1840 = local read "Calibrate:"() -> (w2683:T8)
            n1841 = case shown="\"manipulator 1\", Default" w2683 {
              tunnel: w2680 -> [w2695 w2697 w2699 w2701]
              tunnel: [w2694 w2696 w2698 w2700] -> w2692
              frame "manipulator 1", Default {
                n1842 = Unbundle By Name(w2695) -> ("manip 1"=w2694:refnum<vi>)